vi "HFRR ADV v042.vi"() -> ()   [LabVIEW 2025] (continued)
                n820 = local write "Air Temperature Calibration"(enum32{"True", "Fail"}."Fail" ("Sample Temperature Calibration  2")) -> ()
              }
              frame True {
                n821 = local write "Air Temperature Calibration"(enum32{"True", "Fail"}."True" ("Sample Temperature Calibration  2")) -> ()
                n822 = property on="Accept & Save Air Temperature step 4" class="Bool (strict)"("DisabledEnum"=T19."Enabled" ("Disabled")) -> ()  [unwired: 2 in, 2 out]
              }
            }
          }
          frame #8 {
            # "CAL;END"
          }
          frame #9 {
            n823 = local write "Tab Control 4"(T12."Air Step 4" ("Tab Control 4")) -> ()
          }
        }
      }
      event "Back Stroke step main temperature": Value Change {
        n824 = event-data() -> ()  [unwired: 1 in, 6 out]
        n825 = stacked-sequence {
          frame #0 {
            n826 = Wait (ms)(milliseconds to wait=u32 1000) -> ()  [unwired: 1 out]
          }
          frame #1 {
            # "CAL;END"
            n827 = local write "Due Write"("CAL;END" ("Command")) -> ()
          }
          frame #2 {
            n828 = Wait (ms)(milliseconds to wait=u32 1000) -> ()  [unwired: 1 out]
          }
          frame #3 {
            # "CAL;END"
            n829 = local write "Due Write"("CAL;END" ("Command")) -> ()
          }
          frame #4 {
            n830 = local write "Temperature Selection"(T13."Default" ("Temperature Selection")) -> ()
            n831 = local write "Calibration Selection"(T8."Default" ("Calibration Selection")) -> ()
            n832 = local write "Main Calibration Tab"(T7."Main" ("Main Calibration Tab")) -> ()
            n833 = local write "Tab Control 4"(T12."Main" ("Tab Control 4")) -> ()
          }
        }
      }
      event "TEMPERATURE STEP  Back 4", "TEMPERATURE STEP 1 Back 3", "TEMPERATURE STEP  Back 3", "TEMPERATURE STEP 1 Back 2", "Back Air TEMPERATURE Step 4", "Back SAMPLE TEMPERATURE Step 4": Value Change {
        # "Back Stroke step main temperature"
        n834 = event-data() -> ()  [unwired: 1 in, 6 out]
        n835 = stacked-sequence {
          frame #0 {
            n836 = Wait (ms)(milliseconds to wait=u32 1000) -> ()  [unwired: 1 out]
          }
          frame #1 {
            # "CAL;END"
            n837 = local write "Due Write"("CAL;END" ("Command")) -> ()
          }
          frame #2 {
            n838 = Wait (ms)(milliseconds to wait=u32 1000) -> ()  [unwired: 1 out]
          }
          frame #3 {
            # "CAL;END"
            n839 = local write "Due Write"("CAL;END" ("Command")) -> ()
          }
          frame #4 {
            # "TEMPERATURE STEP  Back 4"
            n840 = local write "Main Calibration Tab"(T7."Temperature" ("Main Calibration Tab")) -> ()
            n841 = local write "Temperature Selection"(T13."Default" ("Temperature Selection")) -> ()
            n842 = local write "Tab Control 4"(T12."Main" ("Tab Control 4")) -> ()
            n843 = local write "Calibration Selection"(T8."Default" ("Calibration Selection")) -> ()
          }
        }
      }
      event "FF BACK", "FF BACK 2", "FF BACK 3", "FF BACK 4", "FF BACK 5", "FF BACK 6", "Accept & Save FF": Value Change {
        n844 = event-data() -> ()  [unwired: 1 in, 6 out]
        n845 = stacked-sequence {
          frame #0 {
            n846 = Wait (ms)(milliseconds to wait=u32 1000) -> ()  [unwired: 1 out]
          }
          frame #1 {
            n847 = local write "Due Write"("VC;0") -> ()
          }
          frame #2 {
            n848 = Wait (ms)(milliseconds to wait=u32 1000) -> ()  [unwired: 1 out]
          }
          frame #3 {
            n849 = local write "Due Write"("VC;0") -> ()
          }
          frame #4 {
            w880 = FALSE
            n850 = local write "FF BACK 2"(w880) -> ()
            n851 = local write "FF BACK 3"(w880) -> ()
            n852 = local write "FF BACK 4"(w880) -> ()
            n853 = local write "FF BACK 5"(w880) -> ()
            n854 = local write "FF BACK 6"(w880) -> ()
            n855 = local write "FF BACK"(w880) -> ()
          }
          frame #5 {
            n856 = local write "Temperature Selection"(T13."Default" ("Temperature Selection")) -> ()
            n857 = local write "Calibration Selection"(T8."Default" ("Calibration Selection")) -> ()
            n858 = local write "Friction Force Tab"(T11."Page 1" ("Friction Force Tab")) -> ()
            n859 = local write "Main Calibration Tab"(T7."Main" ("Main Calibration Tab")) -> ()
          }
        }
      }
      event "FF CONTINUE": Value Change {
        n860 = event-data() -> ()  [unwired: 1 in, 6 out]
        n861 = local write "FF CONTINUE"(FALSE ("FF CONTINUE")) -> ()
        n862 = local write "Friction Force Tab"(T11."Page 2" ("Friction Force Tab")) -> ()
      }
      event "FF CONTINUE 2": Value Change {
        n863 = event-data() -> ()  [unwired: 1 in, 6 out]
        n864 = local write "FF CONTINUE 2"(FALSE ("FF CONTINUE")) -> ()
        n865 = local write "Friction Force Tab"(T11."Page 3" ("Friction Force Tab")) -> ()
      }
      event "FF CONTINUE 3": Value Change {
        n866 = event-data() -> ()  [unwired: 1 in, 6 out]
        n867 = local write "FF CONTINUE 3"(FALSE ("FF CONTINUE")) -> ()
        n868 = local write "Friction Force Tab"(T11."Page 4" ("Friction Force Tab")) -> ()
      }
      event "FF CONTINUE 4": Value Change {
        n869 = event-data() -> ()  [unwired: 1 in, 6 out]
        n870 = local write "FF CONTINUE 4"(FALSE ("FF CONTINUE")) -> ()
        n871 = local write "Friction Force Tab"(T11."Page 5" ("Friction Force Tab")) -> ()
      }
      event "FF CONTINUE 5": Value Change {
        n872 = event-data() -> ()  [unwired: 1 in, 6 out]
        n873 = local write "FF CONTINUE 5"(FALSE ("FF CONTINUE")) -> ()
        n874 = local write "Friction Force Tab"(T11."Page 6" ("Friction Force Tab")) -> ()
      }
      event "Stroke Report Button": Value Change {
        n875 = event-data() -> ()  [unwired: 1 in, 6 out]
        n876 = local read "Point 5 - 1.0 mm"() -> (w896:bool)
        n877 = case shown="False" w896 {
          tunnel: [0.8 1.0] -> w895
          frame False {
          }
          frame True {
          }
        }
        n878 = local read "Machine Serial Number"() -> (w899:string)
        n879 = local read "USERNAME"() -> (w897:string)
        n880 = local write "Stroke Report Button"(FALSE ("Stroke Report Button")) -> ()
        n881 = call "Stroke Calibration Report.vi"("measured_value"=w895, "operator_name"=w897, "Instrument_serial Number"=w899) -> ()  [unwired: 7 in, 2 out]
      }
      event "Sample Report Button": Value Change {
        n882 = event-data() -> ()  [unwired: 1 in, 6 out]
        n883 = local read "Machine Serial Number"() -> (w905:string)
        n884 = local read "Sample 0deg temp"() -> (w902:dbl)
        n885 = local read "Sample 60deg temp"() -> (w903:dbl)
        n886 = local read "USERNAME"() -> (w904:string)
        n887 = call "Temperature Calibration Report.vi"("measured_60"=w903, "measured_zero"=w902, "operator_name"=w904, "Instrument_serial Number"=w905) -> ()  [unwired: 6 in, 2 out]
        n888 = local write "Sample Report Button"(FALSE ("Sample Report Button")) -> ()
      }
      event "Report Button FF": Value Change {
        n889 = event-data() -> ()  [unwired: 1 in, 6 out]
        n890 = local read "FF PASS"() -> (w910:bool)
        n891 = local read "Machine Serial Number"() -> (w913:string)
        n892 = Select(t="PASS", s=w910, f="FAIL") -> (s? t:f=w907:string)
        n893 = local read "USERNAME"() -> (w912:string)
        n894 = call "FF Calibration Report.vi"("pass_or_fail"=w907, "operator_name"=w912, "Instrument_serial Number"=w913) -> ()  [unwired: 7 in, 2 out]
        n895 = local write "Report Button FF"(FALSE ("Sample Report Button")) -> ()
      }
      event "Air Temperature Report Button": Value Change {
        n896 = event-data() -> ()  [unwired: 1 in, 6 out]
        n897 = local read "Machine Serial Number"() -> (w918:string)
        n898 = local read "Air 0deg temp"() -> (w915:dbl)
        n899 = local read "Air 60deg temp"() -> (w916:dbl)
        n900 = local read "USERNAME"() -> (w917:string)
        n901 = call "Air Temperature Calibration Report.vi"("measured_60"=w916, "measured_zero"=w915, "operator_name"=w917, "Instrument_serial Number"=w918) -> ()  [unwired: 6 in, 2 out]
        n902 = local write "Air Temperature Report Button"(FALSE ("Sample Report Button")) -> ()
      }
      event "Quit": Value Change {
        n903 = event-data() -> ()  [unwired: 1 in, 6 out]
      }
    }
    n904 = Wait (ms)(milliseconds to wait=u32 100) -> ()  [unwired: 1 out]
  }
  n905 = while {
    shift-right: [w921] -> _
    shift-left: "Enum - Selector" -> [w922]
    stop <- w923 stop-if-true
    # "Auto Start Logic Loop"
    n906 = case shown="\"Maintain Stage\"" w922 {
      tunnel: [w926 w932 w960 w995 w1024 Auto_Start_enum."Exit" ("Enum - Selector") Auto_Start_enum."Init" ("Enum - Selector")] -> w921
      frame "Init", Default {
        n907 = local read "Auto Start Test"() -> (w925:bool)
        n908 = Select(t=Auto_Start_enum."Humidity & Temperature On" ("Enum - Selector"), s=w925, f=Auto_Start_enum."Init") -> (s? t:f=w926:T15)
      }
      frame "Humidity & Temperature On" {
        n909 = stacked-sequence {
          tunnel: [_ _ _ _ _ _ Auto_Start_enum."Reach point" ("Enum - Selector")] -> w929
          frame #0 {
            w934 = T19."Disabled and Grayed Out" ("Disabled")
            w935 = TRUE ("Heater Button")
            n910 = property on="Humidity" class="Bool (strict)"("DisabledEnum"=w934) -> ()  [unwired: 2 in, 2 out]
            n911 = property on="Heater Button" class="Bool (strict)"("DisabledEnum"=w934) -> ()  [unwired: 2 in, 2 out]
            n912 = local write "Heater Button"(w935) -> ()
            n913 = local write "Humidity"(w935) -> ()
            n914 = property on="Heater Button" class="Bool (strict)"("Val(Sgnl)"=TRUE ("Value (Signaling)")) -> ()  [unwired: 2 in, 2 out]
          }
          frame #1 {
            n915 = Wait (ms)(milliseconds to wait=u32 3000) -> ()  [unwired: 1 out]
          }
          frame #2 {
            n916 = local read "Set Temp"() -> (w941:dbl)
            n917 = Number To Fractional String(number=w941, precision (6)=i16 2) -> (F-format string=w938:string)  [unwired: 2 in]
            n918 = Concatenate Strings("ST;" ("Command"), w938) -> (w939:string)
            n919 = local write "Due Write"(w939) -> ()
          }
          frame #3 {
            n920 = Wait (ms)(milliseconds to wait=u32 1500) -> ()  [unwired: 1 out]
          }
          frame #4 {
            (unwired) i16 2 ("precision (6)")
            n921 = local read "WriteHumidity"() -> (w943:string[])
            n922 = local read "Set Rh"() -> (w946:dbl)
            n923 = Number To Fractional String(number=w946) -> (F-format string=w947:string)  [unwired: 3 in]
            n924 = Concatenate Strings("M;" ("new element/subarray"), w947) -> (w948:string)
            n925 = Insert Into Array(array=w943, new element=w948) -> (w944:string[])  [unwired: 1 in]
            n926 = local write "WriteHumidity"(w944) -> ()
            n927 = local write "Due Write"("HE;1" ("Command")) -> ()
          }
          frame #5 {
            n928 = Wait (ms)(milliseconds to wait=u32 1500) -> ()  [unwired: 1 out]
          }
          frame #6 {
            w951 = TRUE ("Reach point temp")
            n929 = local write "Reach point Humidity"(w951) -> ()
            n930 = local write "Reach point temp"(w951) -> ()
          }
        }
        n931 = local read "Auto Start Test"() -> (w931:bool)
        n932 = Not(x=w931) -> (.not. x?=w930:bool)
        n933 = Select(t=Auto_Start_enum."close", s=w930, f=w929) -> (s? t:f=w932:T15)
      }
      frame "Reach point" {
        w961 = TRUE ("PAUSE")
        w969 = 1.0 ("y")
        w972 = 1.0 ("y")
        n934 = local read "Set Temp"() -> (w954:dbl)
        n935 = local read "Set Humidity:"() -> (w968:dbl)
        n936 = local read "Humidity ( %RH )"() -> (w973:dbl)
        n937 = Add(x=w954, y=w972) -> (x+y=w971:dbl)
        n938 = Subtract(x=w954, y=w972) -> (x-y=w970:dbl)
        n939 = Add(x=w968, y=w969) -> (x+y=w967:dbl)
        n940 = Subtract(x=w968, y=w969) -> (x-y=w966:dbl)
        n941 = local read "TEMP"() -> (w974:dbl)
        n942 = In Range and Coerce(upper limit=w967, x=w973, lower limit=w966) -> (In Range?=w955:bool)  [unwired: 1 out]
        n943 = In Range and Coerce(upper limit=w971, x=w974, lower limit=w970) -> (In Range?=w956:bool)  [unwired: 1 out]
        n944 = disable-structure shown="Enabled" {
          disable-tunnel: w955 -> [w975 _]
          disable-tunnel: [w975 TRUE] -> w953
          frame Disabled {
            n945 = case shown="True" w975 {
              frame False {
              }
              frame True {
                n946 = case shown="True" "Reach point Humidity" {
                  selector: "Reach point Humidity" -> [_ w981]
                  frame False {
                  }
                  frame True {
                    n947 = local read "EVENT LOG"() -> (w978:string)
                    n948 = Not(x=w981) -> (.not. x?=w980:bool)
                    n949 = local write "Reach point Humidity"(w980) -> ()
                    n950 = call "Event Log.vi"("Content"="Target Humidity reached", "EVENT LOG"=w978) -> ("EVENT LOG"=w979:string)  [unwired: 8 in, 1 out]
                    n951 = local write "EVENT LOG"(w979) -> ()
                  }
                }
              }
            }
          }
          frame Enabled {
          }
        }
        n952 = case shown="True" w956 {
          frame False {
          }
          frame True {
            n953 = case shown="True" "Reach point temp" {
              selector: "Reach point temp" -> [_ w988]
              frame False {
              }
              frame True {
                n954 = local read "EVENT LOG"() -> (w985:string)
                n955 = Not(x=w988) -> (.not. x?=w987:bool)
                n956 = local write "Reach point temp"(w987) -> ()
                n957 = call "Event Log.vi"("Content"="Target Temperature reached", "EVENT LOG"=w985) -> ("EVENT LOG"=w986:string)  [unwired: 8 in, 1 out]
                n958 = local write "EVENT LOG"(w986) -> ()
              }
            }
          }
        }
        n959 = local read "Auto Start Test"() -> (w959:bool)
        n960 = And(x=w956, y=w953) -> (x .and. y?=w965:bool)
        n961 = Select(t=Auto_Start_enum."Maintain Stage" ("Enum - Selector"), s=w965, f=Auto_Start_enum."Reach point" ("Enum - Selector")) -> (s? t:f=w962:T15)
        n962 = Not(x=w959) -> (.not. x?=w958:bool)
        n963 = Select(t=Auto_Start_enum."close", s=w958, f=w962) -> (s? t:f=w960:T15)
        n964 = call "ELAPSED TIMER VI.vi"("RESET"=w961, "PAUSE"=w961) -> ()  [unwired: 7 in, 3 out]
      }
      frame "Maintain Stage" {
        w1003 = 2.0 ("y")
        w1002 = 1.0 ("y")
        # "Humidity and temperature set point has stabilized."
        # "Humidity and  temperatures Set Point  have been reached"
        n965 = local read "Set Temp"() -> (w990:dbl)
        n966 = local read "Set Humidity:"() -> (w1006:dbl)
        n967 = local read "Humidity ( %RH )"() -> (w1009:dbl)
        n968 = Add(x=w990, y=w1002) -> (x+y=w1008:dbl)
        n969 = Subtract(x=w990, y=w1002) -> (x-y=w1007:dbl)
        n970 = local read "TEMP"() -> (w1010:dbl)
        n971 = Add(x=w1006, y=w1003) -> (x+y=w1005:dbl)
        n972 = Subtract(x=w1006, y=w1003) -> (x-y=w1004:dbl)
        n973 = In Range and Coerce(upper limit=w1008, x=w1010, lower limit=w1007) -> (In Range?=w1001:bool)  [unwired: 1 out]
        n974 = In Range and Coerce(upper limit=w1005, x=w1009, lower limit=w1004) -> ()  [unwired: 2 out]
        n975 = And(x=w1001, y=TRUE) -> (x .and. y?=w1000:bool)
        n976 = Not(x=w1000) -> (.not. x?=w999:bool)
        n977 = call "ELAPSED TIMER VI.vi"("TARGET"=60.0, "RESET"=w999, "PAUSE"=FALSE) -> ("ELAPSED INDICATION"=w996:bool)  [unwired: 6 in, 2 out]
        n978 = case shown="True" w996 {
          tunnel: w996 -> [_ w1013]
          tunnel: [Auto_Start_enum."Maintain Stage" ("Enum - Selector") w1012] -> w994
          frame False {
          }
          frame True {
            n979 = stacked-sequence {
              tunnel: w1013 -> [_ _ _ _ _]
              tunnel: [_ _ _ _ Auto_Start_enum."Start Stage" ("Enum - Selector")] -> w1012
              frame #0 {
                n980 = local read "EVENT LOG"() -> (w1015:string)
                n981 = call "Event Log.vi"("Content"="Temperature set point has stabilized.", "EVENT LOG"=w1015) -> ("EVENT LOG"=w1016:string)  [unwired: 8 in, 1 out]
                n982 = local write "EVENT LOG"(w1016) -> ()
              }
              frame #1 {
                n983 = Wait (ms)(milliseconds to wait=u32 100) -> ()  [unwired: 1 out]
              }
              frame #2 {
                n984 = local read "EVENT LOG"() -> (w1019:string)
                n985 = call "Event Log.vi"("Content"="Auto Test Started", "EVENT LOG"=w1019) -> ("EVENT LOG"=w1020:string)  [unwired: 8 in, 1 out]
                n986 = local write "EVENT LOG"(w1020) -> ()
              }
              frame #3 {
                w1021 = TRUE ("RUN")
                n987 = local write "RUN"(w1021) -> ()
                n988 = property on="Auto Start Temp" class="Bool (strict)"("Val(Sgnl)"=w1021) -> ()  [unwired: 2 in, 2 out]
                "Auto Start Temp" <- w1021
              }
              frame #4 {
              }
            }
          }
        }
        n989 = local read "Auto Start Test"() -> (w993:bool)
        n990 = Not(x=w993) -> (.not. x?=w992:bool)
        n991 = Select(t=Auto_Start_enum."close", s=w992, f=w994) -> (s? t:f=w995:T15)
      }
      frame "Start Stage" {
        w1023 = TRUE ("PAUSE")
        n992 = local read "Auto Start Test"() -> (w1028:bool)
        n993 = Not(x=w1028) -> (.not. x?=w1027:bool)
        n994 = Select(t=Auto_Start_enum."close" ("Enum - Selector"), s=w1027, f=Auto_Start_enum."Start Stage" ("Enum - Selector")) -> (s? t:f=w1024:T15)
        n995 = call "ELAPSED TIMER VI.vi"("RESET"=w1023, "PAUSE"=w1023) -> ()  [unwired: 7 in, 3 out]
      }
      frame "close" {
        w1031 = FALSE ("Heater Button")
        n996 = local write "RUN"(w1031) -> ()
        n997 = local write "Heater Button"(w1031) -> ()
        n998 = local write "Humidity"(w1031) -> ()
        n999 = local write "Auto Start Test"(w1031) -> ()
        n1000 = property on="Heater Button" class="Bool (strict)"("Val(Sgnl)"=FALSE ("Value (Signaling)")) -> ()  [unwired: 2 in, 2 out]
        n1001 = local write "Humidity 2"(TRUE ("Humidity")) -> ()
      }
      frame "Exit" {
      }
    }
    n1002 = Wait (ms)(milliseconds to wait=u32 100) -> ()  [unwired: 1 out]
    n1003 = local read "Quit"() -> (w923:bool)
  }
  n1004 = property on="Service Password Log" class="Str"("Visible"=w23) -> ()  [unwired: 2 in, 2 out]
  n1005 = property on="Password 3" class="Clust (strict)"("Visible"=w23) -> ()  [unwired: 2 in, 2 out]
  n1006 = while {
    stop <- w1060 stop-if-true
    w1043 = errorcluster {"status"=FALSE, "code"=0, "source"=""} ("error in (no error) 3")
    # "this loop is for manual report generation"
    n1007 = local read "Confirm Measrurement"() -> (w1042:bool)
    n1008 = case shown="True" w1042 {
      selector: w1042 -> [_ w1150]
      tunnel: errorcluster {"status"=FALSE, "code"=0, "source"=""} ("error in (no error) 3") -> [_ w1151]
      tunnel: [_ w1149] -> _
      frame False {
      }
      frame True {
        n1009 = stacked-sequence {
          tunnel: w1151 -> [_ w1184 _]
          tunnel: w1150 -> [_ _ w1291]
          tunnel: [_ w1172 _] -> w1149
          frame #0 {
            n1010 = String To Path(string="C:\\LAB-IQ\\Image Calibrate v01.dcf") -> (path=w1154:path)
            n1011 = Open/Create/Replace File ("Open File")(file path (use dialog)=w1154) -> (refnum out=w1155:refnum<file>)  [unwired: 5 in, 2 out]
            n1012 = for {
              N: 4 -> [_]
              tunnel: w1155 -> [w1161]
              i -> [w1157]
              n1013 = Read from Text File ("Read File")(file (use dialog)=w1161) -> (text=w1162:string)  [unwired: 3 in, 3 out]
              n1014 = String Subset(string=w1162, offset (0)=6, length (rest)=10 ("length (rest)")) -> (substring=w1158:string)
              n1015 = Fract/Exp String To Number(string=w1158) -> (number=w1156:dbl)  [unwired: 3 in, 1 out]
              n1016 = case shown="3" w1157 {
                tunnel: w1156 -> [w1163 w1164 _ w1165 _]
                frame 0 {
                  n1017 = local write "5x Gain"(w1163) -> ()
                }
                frame 1 {
                  n1018 = local write "10x Gain"(w1164) -> ()
                }
                frame 2 {
                }
                frame 3 {
                  n1019 = local write "100x gain"(w1165) -> ()
                }
                frame 4, Default {
                }
              }
            }
          }
          frame #1 {
            n1020 = local read "TEST STANDARD"() -> (w1167:T3)
            n1021 = case shown="\"ISO 12156\"" w1167 {
              tunnel: ["ASTM D6079" "ISO 12156"] -> w1166
              frame "ASTM D6079", Default {
              }
              frame "ISO 12156" {
              }
            }
            n1022 = call "IMAGE ANALYSIS.vi"("Enum"=POST_ANALYSIS_ENUM."GET MEASUREMENTS", "error in"=w1184) -> ("error out"=w1191:errorcluster)  [unwired: 8 in, 1 out]
            n1023 = local read "Magnification :"() -> (w1177:string)
            n1024 = call "Stall Data Flow.vim"("value in"=w1191, "milliseconds to wait"=u32 1000) -> ("value out"=w1190:errorcluster)  [unwired: 1 out]
            n1025 = local read "Test File List :"() -> (w1188:string)
            n1026 = case shown="\"10x\"" w1177 {
              tunnel: [w1227 w1228] -> w1175
              frame "5x", Default {
                n1027 = local read "5x Gain"() -> (w1227:dbl)
              }
              frame "10x" {
                # "5x"
                n1028 = local read "10x Gain"() -> (w1228:dbl)
              }
            }
            n1029 = call "IMAGE ANALYSIS.vi"("Enum"=POST_ANALYSIS_ENUM."READ", "error in"=w1190) -> ("error out"=w1187:errorcluster, "data out"=w1178:string)  [unwired: 8 in]
            n1030 = Match Pattern(string=w1178, regular expression="\"type\": ") -> (after substring=w1182:string)  [unwired: 1 in, 3 out]
            n1031 = call "IMAGE PATH CREATION PY.vi"("error in (no error)"=w1187, "File Name :"=w1188) -> ("error out"=w1186:errorcluster, "File Path"=w1174:path, "File Path String:"=w1169:string)  [unwired: 7 in]
            n1032 = Match Pattern(string=w1182, regular expression=",") -> (before substring=w1168:string)  [unwired: 1 in, 3 out]
            n1033 = local read "Calibration Tab"() -> (w1171:enum32{"Measrument", "Calibrate"})
            n1034 = call "Stall Data Flow.vim"("value in"=w1186, "milliseconds to wait"=u32 250) -> ("value out"=w1170:errorcluster)  [unwired: 1 out]
            n1035 = Equal?(x=w1168, y="\"rectangle\"") -> (x = y?=w1179:bool)
            n1036 = case shown="False" w1179 {
              tunnel: w1178 -> [w1233 w1288]
              tunnel: w1175 -> [_ w1279]
              tunnel: cluster{"major":dbl, "minor":dbl, "average":dbl} {"major"=0.0, "minor"=0.0, "average"=0.0} -> [w1231 w1275]
              tunnel: [w1230 w1272] -> w1173
              tunnel: w1168 -> [w1232 _]
              tunnel: w1175 -> [w1229 _]
              frame False {
                n1037 = Equal?(x=w1232, y="\"line\"") -> (x = y?=w1234:bool)
                n1038 = case shown="True" w1234 {
                  tunnel: w1233 -> [_ w1249]
                  tunnel: w1231 -> [w1236 w1248]
                  tunnel: [w1236 w1246] -> w1230
                  tunnel: w1229 -> [_ w1245]
                  frame False {
                  }
                  frame True {
                    w1244 = 0.0 ("Major Axis")
                    n1039 = Match Pattern(string=w1249, regular expression="\"length_px\":") -> (after substring=w1247:string)  [unwired: 1 in, 3 out]
                    n1040 = property on="Major Axis" class="DigNum (strict)"("Caption.Text"="") -> ()  [unwired: 2 in, 2 out]
                    n1041 = property on="Minor Axis" class="DigNum (strict)"("Caption.Text"="") -> ()  [unwired: 2 in, 2 out]
                    n1042 = property on="Average" class="DigNum (strict)"("Caption.Text"="Line") -> ()  [unwired: 2 in, 2 out]
                    n1043 = Fract/Exp String To Number(string=w1247, default (0 dbl)=0.0 ("default (0 DBL)")) -> (number=w1243:dbl)  [unwired: 2 in, 1 out]
                    "Pixel Value" <- w1243
                    n1044 = Multiply(x=w1243, y=w1245) -> (x*y=w1256:dbl)
                    n1045 = Multiply(x=w1256, y=1000.0) -> (x*y=w1239:dbl)
                    n1046 = Divide(x=w1239, y=1000.0) -> (x/y=w1242:dbl)
                    n1047 = local write "Measurment (mm)"(w1242) -> ()
                    n1048 = Bundle By Name(cluster=w1248, "average"=w1239) -> (w1246:cluster{"major":dbl, "minor":dbl, "average":dbl})
                    n1049 = Number To Fractional String(number=w1239, precision (6)=i16 1) -> (F-format string=w1238:string)  [unwired: 2 in]
                    n1050 = local write "Minor Axis"(w1244) -> ()
                    n1051 = local write "Major Axis"(w1244) -> ()
                    n1052 = Fract/Exp String To Number(string=w1238) -> (number=w1237:dbl)  [unwired: 3 in, 1 out]
                    n1053 = local write "Average"(w1237) -> ()
                  }
                }
              }
              frame True {
                w1276 = 1000.0 ("y")
                w1282 = 0.0 ("default (0 DBL)")
                n1054 = Match Pattern(string=w1288, regular expression=" \"width_px\":") -> (after substring=w1286:string)  [unwired: 1 in, 3 out]
                n1055 = Match Pattern(string=w1286, regular expression="\"height_px\":") -> (before substring=w1284:string, after substring=w1283:string)  [unwired: 1 in, 2 out]
                n1056 = Fract/Exp String To Number(string=w1284, default (0 dbl)=w1282) -> (number=w1281:dbl)  [unwired: 2 in, 1 out]
                n1057 = Fract/Exp String To Number(string=w1283, default (0 dbl)=w1282) -> (number=w1280:dbl)  [unwired: 2 in, 1 out]
                n1058 = Multiply(x=w1281, y=w1279) -> (x*y=w1278:dbl)
                n1059 = Multiply(x=w1280, y=w1279) -> (x*y=w1277:dbl)
                n1060 = Multiply(x=w1278, y=w1276) -> (x*y=w1262:dbl)
                n1061 = Multiply(x=w1277, y=w1276) -> (x*y=w1260:dbl)
                n1062 = Add(x=w1262, y=w1260) -> (x+y=w1274:dbl)
                n1063 = property on="Major Axis" class="DigNum (strict)"("Caption.Text"="Major Axis") -> ()  [unwired: 2 in, 2 out]
                n1064 = property on="Minor Axis" class="DigNum (strict)"("Caption.Text"="Minor Axis") -> ()  [unwired: 2 in, 2 out]
                n1065 = property on="Average" class="DigNum (strict)"("Caption.Text"="Average") -> ()  [unwired: 2 in, 2 out]
                n1066 = Divide(x=w1274, y=2.0) -> (x/y=w1258:dbl)
                n1067 = Bundle By Name(cluster=w1275, "major"=w1262, "minor"=w1260, "average"=w1258) -> (w1272:cluster{"major":dbl, "minor":dbl, "average":dbl})
                n1068 = Number To Fractional String(number=w1260, precision (6)=i16 1) -> (F-format string=w1267:string)  [unwired: 2 in]
                n1069 = Number To Fractional String(number=w1258, precision (6)=i16 1) -> (F-format string=w1268:string)  [unwired: 2 in]
                n1070 = Number To Fractional String(number=w1262, precision (6)=i16 1) -> (F-format string=w1266:string)  [unwired: 2 in]
                n1071 = Fract/Exp String To Number(string=w1267) -> (number=w1259:dbl)  [unwired: 3 in, 1 out]
                n1072 = Fract/Exp String To Number(string=w1268) -> (number=w1257:dbl)  [unwired: 3 in, 1 out]
                n1073 = Fract/Exp String To Number(string=w1266) -> (number=w1261:dbl)  [unwired: 3 in, 1 out]
                n1074 = local write "Major Axis"(w1261) -> ()
                n1075 = local write "Average"(w1257) -> ()
                n1076 = local write "Minor Axis"(w1259) -> ()
              }
            }
            n1077 = case shown="\"Measrument\", Default" w1171 {
              tunnel: w1174 -> [w1201 _]
              tunnel: w1173 -> [w1200 _]
              tunnel: [w1197 w1226] -> w1172
              tunnel: w1170 -> [w1199 w1226]
              tunnel: w1169 -> [w1198 _]
              tunnel: w1166 -> [w1196 _]
              frame "Measrument", Default {
                n1078 = stacked-sequence {
                  tunnel: w1201 -> [w1219 _]
                  tunnel: w1200 -> [w1217 _]
                  tunnel: w1199 -> [w1215 _]
                  tunnel: w1198 -> [w1214 _]
                  tunnel: [w1209 _] -> w1197
                  tunnel: w1196 -> [w1202 _]
                  frame #0 {
                    n1079 = call "IMAGE ANALYSIS.vi"("Enum"=POST_ANALYSIS_ENUM."SAVE IMAGE", "error in"=w1215, "IMAGE FILE PATH"=w1214) -> ("error out"=w1213:errorcluster)  [unwired: 7 in, 1 out]
                    n1080 = call "Stall Data Flow.vim"("value in"=w1213, "milliseconds to wait"=u32 1000) -> ("value out"=w1204:errorcluster)  [unwired: 1 out]
                    n1081 = local read "Test File List :"() -> (w1221:string)
                    n1082 = call "IMAGE ANALYSIS.vi"("Enum"=POST_ANALYSIS_ENUM."MINIMIZE UI", "error in"=w1204) -> ("error out"=w1211:errorcluster)  [unwired: 8 in, 1 out]
                    n1083 = Bundle By Name(cluster=T26 {"File Name"="", "Test Method"="", "Operator"="", "Fuel Description"="", "Date and time"=""} ("Main Ref"), "Test Method"=w1202, "File Name"=w1221) -> (w1222:T26)
                    n1084 = call "Stall Data Flow.vim"("value in"=w1211, "milliseconds to wait"=u32 1500) -> ("value out"=w1206:errorcluster)  [unwired: 1 out]
                    n1085 = call "duf file read.vi"("error in (no error)"=w1206, "Main Ref"=w1222) -> ("error out"=w1220:errorcluster, "Main Ref 2"=w1218:T26)  [unwired: 8 in]
                    n1086 = call "DETECTION REPORT for manual.vi"("error in (no error)"=w1220, "return value 3"=w1217, "Image File Path"=w1219, "Main Ref"=w1218) -> ("error out"=w1216:errorcluster)  [unwired: 7 in]
                    n1087 = call <vilib>:"Clear Errors.vi"("error in (no error)"=w1216) -> ("error out"=w1207:errorcluster)  [unwired: 5 in, 1 out]
                    n1088 = call "IMAGE ANALYSIS.vi"("Enum"=POST_ANALYSIS_ENUM."MINIMIZE UI", "error in"=w1207) -> ("error out"=w1209:errorcluster)  [unwired: 8 in, 1 out]
                  }
                  frame #1 {
                    n1089 = local write "Main Tab"(T2."HOME" ("Main Tab")) -> ()
                    n1090 = local write "Main Dashboard Buttons"(T1."Home" ("Main Dashboard Buttons")) -> ()
                  }
                }
              }
              frame "Calibrate" {
              }
            }
          }
          frame #2 {
            n1091 = Not(x=w1291) -> (.not. x?=w1290:bool)
            n1092 = local write "Confirm Measrurement"(w1290) -> ()
            n1093 = local read "Calibration Tab"() -> (w1289:enum32{"Measrument", "Calibrate"})
            n1094 = case shown="\"Measrument\", Default" w1289 {
              frame "Measrument", Default {
                (unwired) T21."HOME" ("Main Tab")
                n1095 = local write "Main Tab"(T2."HOME" ("Main Tab")) -> ()
              }
              frame "Calibrate" {
              }
            }
          }
        }
      }
    }
    n1096 = local read "Humidity"() -> (w1034:bool)
    n1097 = local read "Save Change"() -> (w1039:bool)
    n1098 = local read "Calibrate"() -> (w1040:bool)
    n1099 = local read "Auto Start Test"() -> (w1035:bool)
    n1100 = case shown="True" w1040 {
      selector: w1040 -> [_ w1147]
      frame False {
      }
      frame True {
        n1101 = Not(x=w1147) -> (.not. x?=w1146:bool)
        n1102 = local write "Calibrate"(w1146) -> ()
        n1103 = local write "Calibration Tab"(enum32{"Measrument", "Calibrate"}."Calibrate" ("Calibration Tab")) -> ()
      }
    }
    n1104 = case shown="True" w1039 {
      selector: w1039 -> [_ w1091]
      frame False {
      }
      frame True {
        n1105 = stacked-sequence {
          tunnel: w1091 -> [_ _ _ _ w1145]
          frame #0 {
            n1106 = call "IMAGE ANALYSIS.vi"("Enum"=POST_ANALYSIS_ENUM."HIDE UI") -> ()  [unwired: 9 in, 2 out]
          }
          frame #1 {
            n1107 = local read "100x gain"() -> (w1093:dbl)
            n1108 = local read "10x Gain"() -> (w1094:dbl)
            n1109 = local read "5x Gain"() -> (w1095:dbl)
            n1110 = Number To Fractional String(number=w1094, width (-)=i16 4, precision (6)=i16 7) -> (F-format string=w1116:string)  [unwired: 1 in]
            n1111 = Number To Fractional String(number=0.0, width (-)=i16 4, precision (6)=i16 7) -> (F-format string=w1111:string)  [unwired: 1 in]
            n1112 = Number To Fractional String(number=w1093, width (-)=i16 4, precision (6)=i16 7) -> (F-format string=w1099:string)  [unwired: 1 in]
            n1113 = Number To Fractional String(number=w1095, width (-)=i16 10 ("precision (6)"), precision (6)=i16 7) -> (F-format string=w1125:string)  [unwired: 1 in]
            n1114 = Concatenate Strings("[CH1]" ("string"), w1125, " - 5x Gain" ("string"), "\r") -> (w1115:string)
            n1115 = Concatenate Strings("[CH2]" ("string"), w1116, " - 10x Gain" ("string"), "\r") -> (w1114:string)
            n1116 = Concatenate Strings("[CH3]" ("string"), w1111, " - 20x Gain" ("string"), "\r") -> (w1105:string)
            n1117 = Concatenate Strings("[CH4]" ("string"), w1099, " - 100x Gain" ("string"), "\r") -> (w1098:string)
            n1118 = String To Path(string="C:\\LAB-IQ\\Image Calibrate v01.dcf") -> (path=w1128:path)
            n1119 = Concatenate Strings(w1115, w1114, w1105, w1098) -> (w1113:string)
            n1120 = call <vilib>:"Write Characters To File.vi"("append to file? (new file:F)"=FALSE, "character string"=w1113, "file path (dialog if empty)"=w1128) -> ()  [unwired: 2 in, 1 out]
          }
          frame #2 {
            n1121 = String To Path(string="C:\\LAB-IQ\\Image Calibrate v01.dcf") -> (path=w1131:path)
            n1122 = Open/Create/Replace File ("Open File")(file path (use dialog)=w1131) -> (refnum out=w1132:refnum<file>)  [unwired: 5 in, 2 out]
            n1123 = for {
              N: 4 -> [_]
              tunnel: w1132 -> [w1138]
              i -> [w1134]
              n1124 = Read from Text File ("Read File")(file (use dialog)=w1138) -> (text=w1139:string)  [unwired: 3 in, 3 out]
              n1125 = String Subset(string=w1139, offset (0)=6, length (rest)=10 ("length (rest)")) -> (substring=w1135:string)
              n1126 = Fract/Exp String To Number(string=w1135) -> (number=w1133:dbl)  [unwired: 3 in, 1 out]
              n1127 = case shown="3" w1134 {
                tunnel: w1133 -> [w1140 w1141 _ w1142 _]
                frame 0 {
                  n1128 = local write "5x Gain"(w1140) -> ()
                }
                frame 1 {
                  n1129 = local write "10x Gain"(w1141) -> ()
                }
                frame 2 {
                }
                frame 3 {
                  n1130 = local write "100x gain"(w1142) -> ()
                }
                frame 4, Default {
                }
              }
            }
          }
          frame #3 {
            n1131 = call "IMAGE ANALYSIS.vi"("Enum"=POST_ANALYSIS_ENUM."SHOW UI") -> ()  [unwired: 9 in, 2 out]
          }
          frame #4 {
            n1132 = Not(x=w1145) -> (.not. x?=w1144:bool)
            n1133 = local write "Save Change"(w1144) -> ()
          }
        }
      }
    }
    n1134 = case shown="False" w1035 {
      tunnel: w1034 -> [w1061 _]
      frame False {
        n1135 = case shown="True" w1061 {
          frame False {
          }
          frame True {
            n1136 = local read "Set Humidity:"() -> (w1065:dbl)
            n1137 = local read "Set Humidity:"() -> (w1068:dbl)
            n1138 = local read "Humidity ( %RH )"() -> (w1069:dbl)
            n1139 = Subtract(x=w1065, y=2.0) -> (x-y=w1063:dbl)
            n1140 = Add(x=w1068, y=2.0) -> (x+y=w1064:dbl)
            n1141 = In Range and Coerce(upper limit=w1064, x=w1069, lower limit=w1063) -> (In Range?=w1062:bool)  [unwired: 1 out]
            n1142 = case shown="True" w1062 {
              frame False {
              }
              frame True {
                n1143 = case shown="True" "Manual Humididty Reached" {
                  selector: "Manual Humididty Reached" -> [_ w1072]
                  frame False {
                  }
                  frame True {
                    n1144 = Not(x=w1072) -> (.not. x?=w1071:bool)
                    n1145 = local write "Manual Humididty Reached"(w1071) -> ()
                    n1146 = local read "EVENT LOG"() -> (w1074:string)
                    n1147 = call "Event Log.vi"("Content"="Target Humidity reached", "EVENT LOG"=w1074) -> ("EVENT LOG"=w1073:string)  [unwired: 8 in, 1 out]
                    n1148 = local write "EVENT LOG"(w1073) -> ()
                  }
                }
              }
            }
          }
        }
      }
      frame True {
        n1149 = local write "Manual Humididty Reached"(TRUE ("Manual Humididty Reached")) -> ()
      }
    }
    n1150 = local read "Cap Live Image"() -> (w1055:bool)
    n1151 = local read "SCAR MEASURMENT"() -> (w1058:enum32{"Auto Scar", "Manual Scar"})
    n1152 = Equal?(x=w1058, y=enum32{"Auto Scar", "Manual Scar"}."Manual Scar" ("SCAR MEASURMENT")) -> (x = y?=w1056:bool)
    n1153 = And(x=w1056, y=w1055) -> (x .and. y?=w1054:bool)
    n1154 = Wait (ms)(milliseconds to wait=u32 250) -> ()  [unwired: 1 out]
    n1155 = case shown="True" w1054 {
      selector: w1054 -> [_ w1377]
      frame False {
      }
      frame True {
        n1156 = stacked-sequence {
          tunnel: [_ _ _ w1396 _] -> _
          tunnel: w1377 -> [_ _ _ _ w1403]
          frame #0 {
            w1378 = 0.0
            n1157 = local write "Major Axis"(w1378) -> ()
            n1158 = local write "Minor Axis"(w1378) -> ()
            n1159 = local write "Average"(w1378) -> ()
          }
          frame #1 {
            n1160 = call "CAMERA LIVE FEED FGV.vi"("Enum - Menu"=CAMERA_LIVE_FEED_ENUM."CAMERA MINIMIZE") -> ()  [unwired: 9 in, 2 out]
          }
          frame #2 {
            n1161 = local read "Magnification len live scar"() -> (w1382:string)
            n1162 = case shown="\"10x\", Default" w1382 {
              tunnel: ["_10x" "_5x"] -> w1381
              frame "10x", Default {
              }
              frame "5x" {
              }
            }
            n1163 = local read "FILE 3"() -> (w1388:string)
            n1164 = call <vilib>:"Trim Whitespace.vi"("string"="C:\\LAB-IQ\\images\\") -> ("trimmed string"=w1390:string)  [unwired: 1 in]
            n1165 = String To Path(string=w1390) -> (path=w1389:path)
            n1166 = Concatenate Strings(w1388, w1381, ".png" ("string")) -> (w1387:string)
            n1167 = Build Path(base path=w1389, name or relative path=w1387) -> (appended path=w1386:path)
            n1168 = Path To String(path=w1386) -> (string=w1385:string)
            n1169 = call "CAMERA LIVE FEED FGV.vi"("Enum - Menu"=CAMERA_LIVE_FEED_ENUM."CAMERA SAVE", "Image Path"=w1385) -> ("error out"=w1383:errorcluster)  [unwired: 8 in, 1 out]
            n1170 = case shown="No Error" w1383 {
              frame No Error {
                n1171 = One Button Dialog(message="Image saved successfully") -> ()  [unwired: 1 in, 1 out]
              }
              frame Error {
              }
            }
          }
          frame #3 {
            n1172 = call "LIST FILE NAMES.vi"() -> ("error out"=w1398:errorcluster, "filenames"=w1395:string[])  [unwired: 10 in]
            n1173 = call "IMAGE ANALYSIS.vi"("Enum"=POST_ANALYSIS_ENUM."SHOW UI", "error in"=w1398) -> ("error out"=w1396:errorcluster)  [unwired: 8 in, 1 out]
            n1174 = property on="Test File List :" class="CmbBox"("Strings[]"=w1395) -> ()  [unwired: 2 in, 2 out]
          }
          frame #4 {
            (unwired) T25."Report" ("Main Dashboard Buttons")
            (unwired) T27."Report" ("Main Dashboard Buttons")
            n1175 = Not(x=w1403) -> (.not. x?=w1402:bool)
            n1176 = local write "Zoom Factore"(0.0 ("Zoom Factore")) -> ()
            n1177 = local write "Cap Live Image"(w1402) -> ()
            n1178 = local write "Main Tab"(T2."Adv Scar Report" ("Main Tab")) -> ()
            n1179 = property on="Cap Live Image" class="Bool (strict)"("BoolText.Text"="Capture Image" ("Boolean Text.Text")) -> ()  [unwired: 2 in, 2 out]
            n1180 = local write "Main Dashboard Buttons"(T1."Report" ("Main Dashboard Buttons")) -> ()
          }
        }
      }
    }
    n1181 = local read "change Gain"() -> (w1038:bool)
    n1182 = local read "Back Square"() -> (w1037:bool)
    n1183 = case shown="True" w1038 {
      selector: w1038 -> [_ w1082]
      frame False {
      }
      frame True {
        n1184 = stacked-sequence {
          tunnel: w1082 -> [_ w1090]
          frame #0 {
            n1185 = local read "Actual (µm)"() -> (w1086:dbl)
            n1186 = local read "Pixel Value"() -> (w1085:dbl)
            n1187 = local read "Magnification :"() -> (w1084:string)
            n1188 = Divide(x=w1086, y=w1085) -> (x/y=w1083:dbl)
            n1189 = case shown="\"10x\"" w1084 {
              tunnel: w1083 -> [w1087 w1088]
              frame "10x" {
                n1190 = local write "10x Gain"(w1087) -> ()
              }
              frame "5x", Default {
                n1191 = local write "5x Gain"(w1088) -> ()
              }
            }
          }
          frame #1 {
            n1192 = Not(x=w1090) -> (.not. x?=w1089:bool)
            n1193 = local write "change Gain"(w1089) -> ()
          }
        }
      }
    }
    n1194 = case shown="True" w1037 {
      selector: w1037 -> [_ w1080]
      frame False {
      }
      frame True {
        n1195 = Not(x=w1080) -> (.not. x?=w1079:bool)
        n1196 = local write "Back Square"(w1079) -> ()
        n1197 = local write "Calibration Tab"(enum32{"Measrument", "Calibrate"}."Measrument" ("Calibration Tab")) -> ()
      }
    }
    n1198 = local read "Rectangle Tool"() -> (w1049:bool)
    n1199 = local read "Clear ROI Tool"() -> (w1048:bool)
    n1200 = local read "Open Image"() -> (w1053:bool)
    n1201 = local read "line tool"() -> (w1050:bool)
    n1202 = local read "OUT"() -> (w1051:bool)
    n1203 = local read "In"() -> (w1052:bool)
    n1204 = case shown="True" w1053 {
      selector: w1053 -> [_ w1363]
      tunnel: [w1354 w1365] -> _
      tunnel: w1043 -> [w1354 w1364]
      frame False {
      }
      frame True {
        w1358 = "_5x" ("regular expression")
        n1205 = Not(x=w1363) -> (.not. x?=w1362:bool)
        n1206 = local write "Open Image"(w1362) -> ()
        n1207 = call "IMAGE ANALYSIS.vi"("Enum"=POST_ANALYSIS_ENUM."HIDE UI", "error in"=w1364) -> ("error out"=w1372:errorcluster)  [unwired: 8 in, 1 out]
        n1208 = call <vilib>:"Clear Errors.vi"("error in (no error)"=w1372) -> ("error out"=w1355:errorcluster)  [unwired: 5 in, 1 out]
        n1209 = call "File Dialog"("start path"=path "C:/LAB-IQ/images", "error in"=w1355) -> ("selected path"=w1357:path, "error out"=w1370:errorcluster)  [unwired: 10 in, 2 out]
        "Image path  2" <- w1357
        n1210 = call <vilib>:"Clear Errors.vi"("error in (no error)"=w1370) -> ("error out"=w1369:errorcluster)  [unwired: 5 in, 1 out]
        n1211 = call "IMAGE ANALYSIS.vi"("Enum"=POST_ANALYSIS_ENUM."OPEN FILE", "error in"=w1369, "File Path"=w1357) -> ("error out"=w1368:errorcluster)  [unwired: 7 in, 1 out]
        n1212 = call <vilib>:"Clear Errors.vi"("error in (no error)"=w1368) -> ("error out"=w1367:errorcluster)  [unwired: 5 in, 1 out]
        n1213 = call "IMAGE ANALYSIS.vi"("Enum"=POST_ANALYSIS_ENUM."SHOW UI", "error in"=w1367) -> ("error out"=w1365:errorcluster)  [unwired: 8 in, 1 out]
        n1214 = local write "Zoom Factore"(100.0 ("Zoom Factore")) -> ()
        n1215 = Strip Path(path=w1357) -> (name=w1360:string)  [unwired: 1 out]
        n1216 = Match Pattern(string=w1360, regular expression=w1358) -> (match substring=w1359:string)  [unwired: 1 in, 3 out]
        n1217 = Equal?(x=w1359, y=w1358) -> (x = y?=w1356:bool)
        n1218 = case shown="False" w1356 {
          frame False {
            n1219 = local write "Magnification :"("10x" ("Magnification :")) -> ()
          }
          frame True {
            n1220 = local write "Magnification :"("5x" ("Magnification :")) -> ()
          }
        }
      }
    }
    n1221 = case shown="True" w1051 {
      selector: w1051 -> [_ w1339]
      tunnel: w1043 -> [w1336 w1344]
      tunnel: [w1336 w1338] -> _
      frame False {
      }
      frame True {
        n1222 = Not(x=w1339) -> (.not. x?=w1337:bool)
        n1223 = local read "Zoom Factore"() -> (w1342:dbl)
        n1224 = local write "OUT"(w1337) -> ()
        n1225 = call "IMAGE ANALYSIS.vi"("Enum"=POST_ANALYSIS_ENUM."ZOOM OUT", "error in"=w1344) -> ("error out"=w1338:errorcluster)  [unwired: 8 in, 1 out]
        n1226 = Divide(x=w1342, y=1.2) -> (x/y=w1340:dbl)
        n1227 = local write "Zoom Factore"(w1340) -> ()
      }
    }
    n1228 = case shown="True" w1052 {
      selector: w1052 -> [_ w1348]
      tunnel: w1043 -> [w1345 w1353]
      tunnel: [w1345 w1346] -> _
      frame False {
      }
      frame True {
        n1229 = Not(x=w1348) -> (.not. x?=w1347:bool)
        n1230 = local read "Zoom Factore"() -> (w1351:dbl)
        n1231 = local write "In"(w1347) -> ()
        n1232 = call "IMAGE ANALYSIS.vi"("Enum"=POST_ANALYSIS_ENUM."ZOOM IN", "error in"=w1353) -> ("error out"=w1346:errorcluster)  [unwired: 8 in, 1 out]
        n1233 = Multiply(x=w1351, y=1.2) -> (x*y=w1349:dbl)
        n1234 = local write "Zoom Factore"(w1349) -> ()
      }
    }
    n1235 = case shown="True" w1048 {
      selector: w1048 -> [_ w1320]
      tunnel: w1043 -> [w1318 w1322]
      tunnel: [w1318 w1321] -> _
      frame False {
      }
      frame True {
        n1236 = Not(x=w1320) -> (.not. x?=w1319:bool)
        n1237 = local write "Clear ROI Tool"(w1319) -> ()
        n1238 = call "IMAGE ANALYSIS.vi"("Enum"=POST_ANALYSIS_ENUM."CLEAR ROI", "error in"=w1322) -> ("error out"=w1321:errorcluster)  [unwired: 8 in, 1 out]
      }
    }
    n1239 = case shown="True" w1050 {
      selector: w1050 -> [_ w1332]
      tunnel: w1043 -> [w1330 w1335]
      tunnel: [w1330 w1333] -> _
      frame False {
      }
      frame True {
        n1240 = Not(x=w1332) -> (.not. x?=w1331:bool)
        n1241 = local write "line tool"(w1331) -> ()
        n1242 = call "IMAGE ANALYSIS.vi"("Enum"=POST_ANALYSIS_ENUM."DRAW LINE", "error in"=w1335) -> ("error out"=w1333:errorcluster)  [unwired: 8 in, 1 out]
      }
    }
    n1243 = case shown="True" w1049 {
      selector: w1049 -> [_ w1326]
      tunnel: w1043 -> [w1324 w1328]
      tunnel: [w1324 w1327] -> _
      frame False {
      }
      frame True {
        n1244 = Not(x=w1326) -> (.not. x?=w1325:bool)
        n1245 = local write "Rectangle Tool"(w1325) -> ()
        n1246 = call "IMAGE ANALYSIS.vi"("Enum"=POST_ANALYSIS_ENUM."DRAW REC", "error in"=w1328) -> ("error out"=w1327:errorcluster)  [unwired: 8 in, 1 out]
      }
    }
    n1247 = local read "SCAR MEASURMENT"() -> (w1036:enum32{"Auto Scar", "Manual Scar"})
    n1248 = local read "Fit to Screen Tool"() -> (w1045:bool)
    n1249 = local read "Resize Tool"() -> (w1044:bool)
    n1250 = case shown="\"Manual Scar\", Default" w1036 {
      frame "Auto Scar" {
        n1251 = property on="Cap Live Image" class="Bool (strict)"("BoolText.Text"="Report" ("Boolean Text.Text")) -> ()  [unwired: 2 in, 2 out]
      }
      frame "Manual Scar", Default {
        n1252 = property on="Cap Live Image" class="Bool (strict)"("BoolText.Text"="Save Image" ("Boolean Text.Text")) -> ()  [unwired: 2 in, 2 out]
      }
    }
    n1253 = local read "ROI Color Tool"() -> (w1046:bool)
    n1254 = local read "Pan Tool"() -> (w1047:bool)
    n1255 = case shown="True" w1047 {
      selector: w1047 -> [_ w1314]
      tunnel: w1043 -> [w1312 w1316]
      tunnel: [w1312 w1315] -> _
      frame False {
      }
      frame True {
        n1256 = Not(x=w1314) -> (.not. x?=w1313:bool)
        n1257 = call "IMAGE ANALYSIS.vi"("Enum"=POST_ANALYSIS_ENUM."PAN", "error in"=w1316) -> ("error out"=w1315:errorcluster)  [unwired: 8 in, 1 out]
        n1258 = local write "Pan Tool"(w1313) -> ()
      }
    }
    n1259 = case shown="True" w1044 {
      selector: w1044 -> [_ w1298]
      tunnel: w1043 -> [w1293 w1295]
      tunnel: [w1293 w1294] -> _
      frame False {
      }
      frame True {
        n1260 = Not(x=w1298) -> (.not. x?=w1297:bool)
        n1261 = local write "Resize Tool"(w1297) -> ()
        n1262 = call "IMAGE ANALYSIS.vi"("Enum"=POST_ANALYSIS_ENUM."RESIZE MODE", "error in"=w1295) -> ("error out"=w1294:errorcluster)  [unwired: 8 in, 1 out]
      }
    }
    n1263 = case shown="True" w1045 {
      selector: w1045 -> [_ w1303]
      tunnel: [w1299 w1304] -> _
      tunnel: w1043 -> [w1299 w1302]
      frame False {
      }
      frame True {
        n1264 = Not(x=w1303) -> (.not. x?=w1301:bool)
        n1265 = local write "Zoom Factore"(100.0 ("Zoom Factore")) -> ()
        n1266 = local write "Fit to Screen Tool"(w1301) -> ()
        n1267 = call "IMAGE ANALYSIS.vi"("Enum"=POST_ANALYSIS_ENUM."FIT", "error in"=w1302) -> ("error out"=w1304:errorcluster)  [unwired: 8 in, 1 out]
      }
    }
    n1268 = case shown="True" w1046 {
      selector: w1046 -> [_ w1309]
      tunnel: [w1306 w1310] -> _
      tunnel: w1043 -> [w1306 w1307]
      frame False {
      }
      frame True {
        n1269 = Not(x=w1309) -> (.not. x?=w1308:bool)
        n1270 = local write "ROI Color Tool"(w1308) -> ()
        n1271 = call "IMAGE ANALYSIS.vi"("Enum"=POST_ANALYSIS_ENUM."SET ROI COLOR", "error in"=w1307) -> ("error out"=w1310:errorcluster)  [unwired: 8 in, 1 out]
      }
    }
    n1272 = local read "Quit"() -> (w1060:bool)
  }
  n1273 = while {
    stop <- w1405 stop-if-true
    n1274 = local read "Image Path"() -> (w1408:path)
    n1275 = local read "Print 3"() -> (w1411:bool)
    n1276 = Equal?(x=w1408, y=path "") -> (x = y?=w1407:bool)
    n1277 = Not(x=w1407) -> (.not. x?=w1406:bool)
    n1278 = property on="Print 3" class="Bool (strict)"("Visible"=w1406) -> ()  [unwired: 2 in, 2 out]
    n1279 = case shown="True" w1411 {
      frame False {
        n1280 = local write "Rd"(TRUE ("Boolean 7")) -> ()
      }
      frame True {
        n1281 = flat-sequence {
          tunnel: [w1451] -> w1419
          tunnel: [w1438] -> w1417
          tunnel: [w1448] -> w1413
          tunnel: w1419 -> [w1460]
          tunnel: [w1460] -> w1418
          tunnel: w1417 -> [w1459]
          tunnel: [w1459] -> w1416
          tunnel: [w1457] -> w1415
          tunnel: [w1456] -> w1414
          tunnel: w1413 -> [w1456]
          tunnel: w1418 -> [w1462]
          tunnel: w1416 -> [w1463]
          tunnel: w1415 -> [_]
          tunnel: w1414 -> [w1461]
          frame #0 {
            n1282 = case shown="True" "Rd" {
              frame False {
              }
              frame True {
                n1283 = while {
                  tunnel: "abcdefABCDEF" ("string 2") -> [w1430]
                  shift-right: [w1428] -> w1422
                  shift-left: "" -> [w1427]
                  i -> [w1437]
                  stop <- w1436 stop-if-true
                  n1284 = Random Number (0-1)() -> (number: 0 to 1=w1431:dbl)
                  n1285 = Multiply(x=w1431, y=62.0) -> (x*y=w1433:dbl)
                  n1286 = Decrement(x="Length 2") -> (x-1=w1426:i16)
                  n1287 = To Word Integer(number=w1433) -> (16bit integer=w1434:i16)
                  n1288 = String Subset(string=w1430, offset (0)=w1434, length (rest)=1 ("length (rest)")) -> (substring=w1429:string)
                  n1289 = Greater Or Equal?(x=w1437, y=w1426) -> (x >= y?=w1436:bool)
                  n1290 = Concatenate Strings(w1429, w1427) -> (w1428:string)
                }
                "String 10" <- w1422
                n1291 = local write "Rd"(FALSE ("Boolean 7")) -> ()
              }
            }
          }
          frame #1 {
            w1449 = "_resized.jpg" ("command line")
            (unwired) ".jpg -resize 320x240 " ("string")
            (unwired) "Choose an Image File" ("prompt")
            # "-resize 1798x425"
            n1292 = local read "Image Path"() -> (w1443:path)
            n1293 = Strip Path(path=w1443) -> (stripped path=w1438:path, name=w1439:string)
            n1294 = Match Pattern(string=w1439, regular expression=".jpg") -> (before substring=→"before substring 2":string, after substring=→"after substring":string)  [unwired: 1 in, 2 out]
            n1295 = Match Pattern(string=w1439, regular expression="\\") -> (before substring=w1445:string)  [unwired: 1 in, 3 out]
            n1296 = Match Pattern(string=w1445, regular expression=".jpg") -> (before substring=w1444:string)  [unwired: 1 in, 3 out]
            n1297 = Concatenate Strings("cmd /c convert " ("string"), w1444, ".jpg -resize 320x240  " ("command line"), w1444, w1449) -> (w1452:string)
            n1298 = call <vilib>:"System Exec.vi"("run minimized? (F)"=TRUE, "wait until completion? (T)"=TRUE, "working directory"=w1438, "command line"=w1452) -> ("error out"=w1451:errorcluster)  [unwired: 4 in, 3 out]
            "error out 2" <- w1451
            n1299 = Concatenate Strings(w1444, w1449) -> (w1448:string)
          }
          frame #2 {
            n1300 = Wait (ms)(milliseconds to wait=u32 2000 ("millisecond timer value")) -> (millisecond timer value=w1457:u32)
          }
          frame #3 {
            n1301 = case shown="No Error" w1462 {
              tunnel: w1463 -> [w1466 _]
              tunnel: w1461 -> [w1464 _]
              frame No Error {
                (unwired) ".jpg" ("string")
                n1302 = Path To String(path=w1466) -> (string=w1470:string)
                n1303 = Concatenate Strings(w1470, "\\" ("string"), w1464) -> (w1469:string)
                n1304 = String To Path(string=w1469) -> (path=w1468:path)
                n1305 = call <vilib>:"Read JPEG File.vi"("path to JPEG file"=w1468) -> ("image data"=w1472:T16)  [unwired: 8 in, 2 out]
                "image data" <- w1472
                n1306 = local write "Print 3"(FALSE ("Print 2")) -> ()
                n1307 = call <vilib>:"Draw Flattened Pixmap.vi"("image data"=w1472) -> ("new picture"=→"new picture":picture)  [unwired: 8 in]
              }
              frame Error {
              }
            }
          }
        }
      }
    }
    n1308 = Wait (ms)(milliseconds to wait=u32 20 ("millisecond timer value")) -> ()  [unwired: 1 out]
    n1309 = local read "Quit"() -> (w1405:bool)
  }
  n1310 = while {
    tunnel: w40 -> [_]
    tunnel: w26 -> [_]
    stop <- w1502 stop-if-true
    # "New Adv Logics"
    n1311 = local read "Main Tab"() -> (w1483:T2)
    n1312 = local read "Main Tab"() -> (w1500:T2)
    n1313 = local read "Sign In"() -> (w1499:bool)
    n1314 = case shown="\"Adv Scar\"" w1483 {
      frame "HOME", Default {
        n1315 = local read "LIVE FEED MIN TEMP"() -> (w1635:bool)
        n1316 = local write "LIVE FEED MAX TEMP"(TRUE ("LIVE FEED MAX TEMP")) -> ()
        n1317 = local read "CAMERA ROI MIN TEMP"() -> (w1633:bool)
        n1318 = case shown="True" w1635 {
          selector: w1635 -> [_ w1642]
          frame False {
          }
          frame True {
            n1319 = Not(x=w1642) -> (.not. x?=w1641:bool)
            n1320 = local write "LIVE FEED MIN TEMP"(w1641) -> ()
            n1321 = call "CAMERA LIVE FEED FGV.vi"("Enum - Menu"=CAMERA_LIVE_FEED_ENUM."CAMERA MINIMIZE") -> ()  [unwired: 9 in, 2 out]
          }
        }
        n1322 = case shown="True" w1633 {
          selector: w1633 -> [_ w1639]
          frame False {
          }
          frame True {
            n1323 = Not(x=w1639) -> (.not. x?=w1638:bool)
            n1324 = local write "CAMERA ROI MIN TEMP"(w1638) -> ()
            n1325 = call "IMAGE ANALYSIS.vi"("Enum"=POST_ANALYSIS_ENUM."MINIMIZE UI") -> ()  [unwired: 9 in, 2 out]
          }
        }
        n1326 = local write "CAMERA ROI MAX TEMP"(TRUE ("CAMERA ROI MAX TEMP")) -> ()
      }
      frame "Test Setup" {
        n1327 = local read "LIVE FEED MIN TEMP"() -> (w1645:bool)
        n1328 = local read "CAMERA ROI MIN TEMP"() -> (w1643:bool)
        n1329 = local write "LIVE FEED MAX TEMP"(TRUE ("LIVE FEED MAX TEMP")) -> ()
        n1330 = case shown="True" w1645 {
          selector: w1645 -> [_ w1652]
          frame False {
          }
          frame True {
            n1331 = Not(x=w1652) -> (.not. x?=w1651:bool)
            n1332 = local write "LIVE FEED MIN TEMP"(w1651) -> ()
            n1333 = call "CAMERA LIVE FEED FGV.vi"("Enum - Menu"=CAMERA_LIVE_FEED_ENUM."CAMERA MINIMIZE") -> ()  [unwired: 9 in, 2 out]
          }
        }
        n1334 = case shown="True" w1643 {
          selector: w1643 -> [_ w1649]
          frame False {
          }
          frame True {
            n1335 = Not(x=w1649) -> (.not. x?=w1648:bool)
            n1336 = local write "CAMERA ROI MIN TEMP"(w1648) -> ()
            n1337 = call "IMAGE ANALYSIS.vi"("Enum"=POST_ANALYSIS_ENUM."MINIMIZE UI") -> ()  [unwired: 9 in, 2 out]
          }
        }
        n1338 = local write "CAMERA ROI MAX TEMP"(TRUE ("CAMERA ROI MAX TEMP")) -> ()
      }
      frame "Acquire" {
        n1339 = local read "LIVE FEED MIN TEMP"() -> (w1655:bool)
        n1340 = local write "LIVE FEED MAX TEMP"(TRUE ("LIVE FEED MAX TEMP")) -> ()
        n1341 = local read "CAMERA ROI MIN TEMP"() -> (w1653:bool)